vi "FlexMag - 23-03-2023.vi"() -> ()   [LabVIEW 2018] (continued)
            # "Cheksum 3 haneli olmalı"
            # "Address"
            n5110 = Concatenate Strings("003" ("write buffer"), "10" ("string"), "010" ("string"), "06" ("string"), "000000" ("string")) -> (w9122:string)
            n5111 = String To Byte Array(string=w9122) -> (unsigned byte array=w9127:u8[])
            n5112 = for {
              tunnel: w9127 -> [w9148] mode=indexing
              shift-right: [w9146] -> w9129
              shift-left: u8 0 -> [w9147]
              n5113 = Add(x=w9148, y=w9147) -> (x+y=w9146:u8)
            }
            n5114 = Number To Decimal String(number=w9129) -> (decimal integer string=w9124:string)  [unwired: 1 in]
            n5115 = local write "Tp3 auto stop"(FALSE ("Tp3_auto_stop")) -> ()
            n5116 = String Length(string=w9124) -> (length=w9125:i32)
            n5117 = case shown="0, Default" w9125 {
              tunnel: w9124 -> [_ w9141 w9144 w9145]
              tunnel: ["" w9139 w9142 w9145] -> w9123
              frame 0, Default {
              }
              frame 1 {
                n5118 = Concatenate Strings("00" ("string"), w9141) -> (w9139:string)
              }
              frame 2 {
                n5119 = Concatenate Strings("0" ("string"), w9144) -> (w9142:string)
              }
              frame 3 {
              }
            }
            n5120 = Concatenate Strings(w9122, w9123, "\r") -> (w9119:string)
            n5121 = VISA Write(VISA resource name=w9118, write buffer=w9119, error in (no error)=w9117) -> (VISA resource name out=w9121:refnum<visa-resource-name>, error out=w9120:errorcluster)  [unwired: 1 out]
            n5122 = stacked-sequence {
              tunnel: [w9137] -> w9114
              tunnel: w9121 -> [w9137]
              tunnel: [w9136] -> w9113
              tunnel: w9120 -> [w9136]
              frame #0 {
                n5123 = Wait (ms)(milliseconds to wait=u32 100) -> ()  [unwired: 1 out]
              }
            }
            "Tp3_stop_cmnd" <- TRUE ("Tp3_stop_cmnd")
          }
          frame 3 {
            # "Cheksum 3 haneli olmalı"
            # "Address"
            n5124 = Multiply(x="Low_speed_value 3", y=ext 10.0) -> (x*y=w9156:ext)
            n5125 = To Unsigned Long Integer(number=w9156) -> (unsigned 32bit integer=w9155:u32)
            n5126 = Number To Decimal String(number=w9155) -> (decimal integer string=w9153:string)  [unwired: 1 out]
            n5127 = String Length(string=w9153) -> (length=w9154:i32)
            n5128 = case shown="0, Default" w9154 {
              tunnel: w9153 -> [_ w9180 w9183 w9184]
              tunnel: ["" w9179 w9182 w9184] -> w9152
              frame 0, Default {
              }
              frame 1 {
                n5129 = Concatenate Strings(w9180, "00" ("string")) -> (w9179:string)
              }
              frame 2 {
                n5130 = Concatenate Strings(w9183, "0" ("string")) -> (w9182:string)
              }
              frame 3 {
              }
            }
            n5131 = Concatenate Strings("003" ("write buffer"), "10" ("string"), "707" ("string"), "06" ("string"), "00" ("string"), w9152) -> (w9164:string)
            n5132 = String To Byte Array(string=w9164) -> (unsigned byte array=w9169:u8[])
            n5133 = for {
              tunnel: w9169 -> [w9198] mode=indexing
              shift-right: [w9196] -> w9171
              shift-left: u8 0 -> [w9197]
              n5134 = Add(x=w9198, y=w9197) -> (x+y=w9196:u8)
            }
            n5135 = Number To Decimal String(number=w9171) -> (decimal integer string=w9166:string)  [unwired: 1 in]
            n5136 = String Length(string=w9166) -> (length=w9167:i32)
            n5137 = case shown="0, Default" w9167 {
              tunnel: w9166 -> [_ w9191 w9194 w9195]
              tunnel: ["" w9189 w9192 w9195] -> w9165
              frame 0, Default {
              }
              frame 1 {
                n5138 = Concatenate Strings("00" ("string"), w9191) -> (w9189:string)
              }
              frame 2 {
                n5139 = Concatenate Strings("0" ("string"), w9194) -> (w9192:string)
              }
              frame 3 {
              }
            }
            n5140 = Concatenate Strings(w9164, w9165, "\r") -> (w9161:string)
            n5141 = VISA Write(VISA resource name=w9160, write buffer=w9161, error in (no error)=w9159) -> (VISA resource name out=w9163:refnum<visa-resource-name>, error out=w9162:errorcluster)  [unwired: 1 out]
            n5142 = local write "Tp3 auto set speed"(FALSE ("Tp3_auto_set_speed")) -> ()
            n5143 = stacked-sequence {
              tunnel: [w9187] -> w9151
              tunnel: w9163 -> [w9187]
              tunnel: [w9186] -> w9150
              tunnel: w9162 -> [w9186]
              frame #0 {
                n5144 = Wait (ms)(milliseconds to wait=u32 100) -> ()  [unwired: 1 out]
              }
            }
          }
          frame 4 {
            # "Cheksum 3 haneli olmalı"
            # "Address"
            n5145 = Concatenate Strings("003" ("write buffer"), "10" ("string"), "026" ("string"), "03" ("string"), "001" ("string")) -> (w9207:string)
            n5146 = String To Byte Array(string=w9207) -> (unsigned byte array=w9212:u8[])
            n5147 = for {
              tunnel: w9212 -> [w9233] mode=indexing
              shift-right: [w9231] -> w9214
              shift-left: u8 0 -> [w9232]
              n5148 = Add(x=w9233, y=w9232) -> (x+y=w9231:u8)
            }
            n5149 = Number To Decimal String(number=w9214) -> (decimal integer string=w9209:string)  [unwired: 1 in]
            n5150 = String Length(string=w9209) -> (length=w9210:i32)
            n5151 = case shown="0, Default" w9210 {
              tunnel: w9209 -> [_ w9226 w9229 w9230]
              tunnel: ["" w9224 w9227 w9230] -> w9208
              frame 0, Default {
              }
              frame 1 {
                n5152 = Concatenate Strings("00" ("string"), w9226) -> (w9224:string)
              }
              frame 2 {
                n5153 = Concatenate Strings("0" ("string"), w9229) -> (w9227:string)
              }
              frame 3 {
              }
            }
            n5154 = local write "Tp3 auto low speed"(FALSE) -> ()
            n5155 = Concatenate Strings(w9207, w9208, "\r") -> (w9204:string)
            n5156 = VISA Write(VISA resource name=w9203, write buffer=w9204, error in (no error)=w9202) -> (VISA resource name out=w9206:refnum<visa-resource-name>, error out=w9205:errorcluster)  [unwired: 1 out]
            n5157 = stacked-sequence {
              tunnel: [w9222] -> w9201
              tunnel: w9206 -> [w9222]
              tunnel: [w9221] -> w9200
              tunnel: w9205 -> [w9221]
              frame #0 {
                n5158 = Wait (ms)(milliseconds to wait=u32 100) -> ()  [unwired: 1 out]
              }
            }
          }
          frame 5 {
            # "Cheksum 3 haneli olmalı"
            # "Address"
            n5159 = Concatenate Strings("003" ("write buffer"), "10" ("string"), "026" ("string"), "03" ("string"), "000" ("string")) -> (w9242:string)
            n5160 = String To Byte Array(string=w9242) -> (unsigned byte array=w9247:u8[])
            n5161 = for {
              tunnel: w9247 -> [w9268] mode=indexing
              shift-right: [w9266] -> w9249
              shift-left: u8 0 -> [w9267]
              n5162 = Add(x=w9268, y=w9267) -> (x+y=w9266:u8)
            }
            n5163 = local write "Tp3 auto normal speed"(FALSE ("Tp3_auto_normal_speed")) -> ()
            n5164 = Number To Decimal String(number=w9249) -> (decimal integer string=w9244:string)  [unwired: 1 in]
            n5165 = String Length(string=w9244) -> (length=w9245:i32)
            n5166 = case shown="0, Default" w9245 {
              tunnel: w9244 -> [_ w9261 w9264 w9265]
              tunnel: ["" w9259 w9262 w9265] -> w9243
              frame 0, Default {
              }
              frame 1 {
                n5167 = Concatenate Strings("00" ("string"), w9261) -> (w9259:string)
              }
              frame 2 {
                n5168 = Concatenate Strings("0" ("string"), w9264) -> (w9262:string)
              }
              frame 3 {
              }
            }
            n5169 = Concatenate Strings(w9242, w9243, "\r") -> (w9239:string)
            n5170 = VISA Write(VISA resource name=w9238, write buffer=w9239, error in (no error)=w9237) -> (VISA resource name out=w9241:refnum<visa-resource-name>, error out=w9240:errorcluster)  [unwired: 1 out]
            n5171 = stacked-sequence {
              tunnel: [w9257] -> w9236
              tunnel: w9241 -> [w9257]
              tunnel: [w9256] -> w9235
              tunnel: w9240 -> [w9256]
              frame #0 {
                n5172 = Wait (ms)(milliseconds to wait=u32 100) -> ()  [unwired: 1 out]
              }
            }
          }
          frame 6 {
            # "Cheksum 3 haneli olmalı"
            # "Address"
            n5173 = Concatenate Strings("003" ("write buffer"), "10" ("string"), "023" ("string"), "06" ("string"), "111111" ("string")) -> (w9276:string)
            n5174 = String To Byte Array(string=w9276) -> (unsigned byte array=w9281:u8[])
            n5175 = for {
              tunnel: w9281 -> [w9302] mode=indexing
              shift-right: [w9300] -> w9283
              shift-left: u8 0 -> [w9301]
              n5176 = Add(x=w9302, y=w9301) -> (x+y=w9300:u8)
            }
            n5177 = Number To Decimal String(number=w9283) -> (decimal integer string=w9278:string)  [unwired: 1 in]
            n5178 = String Length(string=w9278) -> (length=w9279:i32)
            n5179 = case shown="0, Default" w9279 {
              tunnel: w9278 -> [_ w9295 w9298 w9299]
              tunnel: ["" w9293 w9296 w9299] -> w9277
              frame 0, Default {
              }
              frame 1 {
                n5180 = Concatenate Strings("00" ("string"), w9295) -> (w9293:string)
              }
              frame 2 {
                n5181 = Concatenate Strings("0" ("string"), w9298) -> (w9296:string)
              }
              frame 3 {
              }
            }
            n5182 = Concatenate Strings(w9276, w9277, "\r") -> (w9273:string)
            n5183 = VISA Write(VISA resource name=w9272, write buffer=w9273, error in (no error)=w9271) -> (VISA resource name out=w9275:refnum<visa-resource-name>, error out=w9274:errorcluster)  [unwired: 1 out]
            n5184 = stacked-sequence {
              tunnel: [w9291] -> w9270
              tunnel: w9275 -> [w9291]
              tunnel: [w9290] -> w9269
              tunnel: w9274 -> [w9290]
              frame #0 {
                n5185 = Wait (ms)(milliseconds to wait=u32 100) -> ()  [unwired: 1 out]
              }
            }
          }
          frame 7 {
            # "Cheksum 3 haneli olmalı"
            # "Address"
            n5186 = Concatenate Strings("003" ("write buffer"), "10" ("string"), "023" ("string"), "06" ("string"), "000000" ("string")) -> (w9310:string)
            n5187 = String To Byte Array(string=w9310) -> (unsigned byte array=w9315:u8[])
            n5188 = for {
              tunnel: w9315 -> [w9336] mode=indexing
              shift-right: [w9334] -> w9317
              shift-left: u8 0 -> [w9335]
              n5189 = Add(x=w9336, y=w9335) -> (x+y=w9334:u8)
            }
            n5190 = Number To Decimal String(number=w9317) -> (decimal integer string=w9312:string)  [unwired: 1 in]
            n5191 = String Length(string=w9312) -> (length=w9313:i32)
            n5192 = case shown="0, Default" w9313 {
              tunnel: w9312 -> [_ w9329 w9332 w9333]
              tunnel: ["" w9327 w9330 w9333] -> w9311
              frame 0, Default {
              }
              frame 1 {
                n5193 = Concatenate Strings("00" ("string"), w9329) -> (w9327:string)
              }
              frame 2 {
                n5194 = Concatenate Strings("0" ("string"), w9332) -> (w9330:string)
              }
              frame 3 {
              }
            }
            n5195 = Concatenate Strings(w9310, w9311, "\r") -> (w9307:string)
            n5196 = VISA Write(VISA resource name=w9306, write buffer=w9307, error in (no error)=w9305) -> (VISA resource name out=w9309:refnum<visa-resource-name>, error out=w9308:errorcluster)  [unwired: 1 out]
            n5197 = stacked-sequence {
              tunnel: [w9325] -> w9304
              tunnel: w9309 -> [w9325]
              tunnel: [w9324] -> w9303
              tunnel: w9308 -> [w9324]
              frame #0 {
                n5198 = Wait (ms)(milliseconds to wait=u32 100) -> ()  [unwired: 1 out]
              }
            }
          }
        }
      }
      frame #3 {
        n5199 = Or(x="Tp4 low speed gui", y="Tp4 auto low speed") -> (x .or. y?=w9351:bool)
        n5200 = Or(x="Tp4 set speed gui", y="Tp4 auto set speed") -> (x .or. y?=w9354:bool)
        n5201 = Or(x="Tp4 normal speed gui", y="Tp4 auto normal speed") -> (x .or. y?=w9348:bool)
        n5202 = Compound Arithmetic op=OR("Tp4 stop gui", "Tp4 stop gui 1", "Tp4 auto stop") -> (w9339:bool)
        n5203 = Compound Arithmetic op=OR("Tp4 start gui", "Tp4 start gui 1", "Tp4 auto start") -> (w9338:bool)
        n5204 = case shown="True" w9338 {
          tunnel: [FALSE w9367] -> w9337
          frame False {
          }
          frame True {
            n5205 = case shown="False" "tp4 start safety" {
              tunnel: [FALSE TRUE] -> w9367
              frame False {
                n5206 = local write "Tp4 auto start"(FALSE ("Tp1_auto_start")) -> ()
                n5207 = local write "Warning Message"("CH4 TP cannot be started." ("Error Message")) -> ()
              }
              frame True {
              }
            }
          }
        }
        n5208 = Build Array(FALSE, w9337, w9339, w9354, w9351, w9348, "Tp4 start initial", "Tp4 stop initial") -> (w9358:bool[])
        n5209 = Boolean Array To Number(Boolean array=w9358) -> (number=w9364:u32)
        n5210 = Mantissa & Exponent(0:w9364) -> (2:w9363:dbl)  [unwired: 1 out]
        n5211 = case shown="0, Default" w9363 {
          tunnel: w9362 -> [w9372 w9487 w9523 w9565 w9608 w9643 w9677 w9711]
          tunnel: w9361 -> [w9373 w9486 w9522 w9564 w9607 w9642 w9676 w9710]
          tunnel: [w9375 w9485 w9521 w9563 w9606 w9641 w9675 w9709] -> w9360
          tunnel: [w9374 w9484 w9520 w9562 w9605 w9640 w9674 w9708] -> w9359
          frame 0, Default {
            n5212 = stacked-sequence {
              seq-local: [w9381 _] -> [_ w9439]
              seq-local: [w9380 _] -> [_ w9440]
              tunnel: w9372 -> [w9391 _]
              tunnel: w9373 -> [w9390 _]
              tunnel: [_ w9442] -> w9375
              tunnel: [_ w9441] -> w9374
              frame #0 {
                # "Address"
                # "Cheksum 3 haneli olmalı"
                # "Address"
                n5213 = Concatenate Strings("004" ("write buffer"), "00" ("string"), "309" ("string"), "02" ("string"), "=?" ("string")) -> (w9400:string)
                n5214 = String To Byte Array(string=w9400) -> (unsigned byte array=w9405:u8[])
                n5215 = for {
                  tunnel: w9405 -> [w9437] mode=indexing
                  shift-right: [w9435] -> w9407
                  shift-left: u8 0 -> [w9436]
                  n5216 = Add(x=w9437, y=w9436) -> (x+y=w9435:u8)
                }
                n5217 = Number To Decimal String(number=w9407) -> (decimal integer string=w9402:string)  [unwired: 1 in]
                n5218 = String Length(string=w9402) -> (length=w9403:i32)
                n5219 = case shown="0, Default" w9403 {
                  tunnel: w9402 -> [_ w9430 w9433 w9434]
                  tunnel: ["" w9428 w9431 w9434] -> w9401
                  frame 0, Default {
                  }
                  frame 1 {
                    n5220 = Concatenate Strings("00" ("string"), w9430) -> (w9428:string)
                  }
                  frame 2 {
                    n5221 = Concatenate Strings("0" ("string"), w9433) -> (w9431:string)
                  }
                  frame 3 {
                  }
                }
                n5222 = Concatenate Strings(w9400, w9401, "\r") -> (w9392:string)
                n5223 = VISA Write(VISA resource name=w9391, write buffer=w9392, error in (no error)=w9390) -> (VISA resource name out=w9395:refnum<visa-resource-name>, error out=w9394:errorcluster)  [unwired: 1 out]
                n5224 = stacked-sequence {
                  tunnel: [w9426] -> w9397
                  tunnel: w9395 -> [w9426]
                  tunnel: [w9425] -> w9396
                  tunnel: w9394 -> [w9425]
                  frame #0 {
                    n5225 = Wait (ms)(milliseconds to wait=u32 100) -> ()  [unwired: 1 out]
                  }
                }
                n5226 = property class="Instr"(reference=w9397, error in=w9396) -> (reference out=w9399:refnum<visa-resource-name>, error out=w9398:errorcluster, "Serial Settings:Number of Bytes at Serial Port"=w9393:u32)
                n5227 = VISA Read(VISA resource name=w9399, byte count=w9393, error in (no error)=w9398) -> (VISA resource name out=w9381:refnum<visa-resource-name>, read buffer=w9388:string, error out=w9380:errorcluster)  [unwired: 1 out]
                n5228 = String Length(string=w9388) -> (length=w9389:i32)
                n5229 = Not Equal To 0?(x=w9389) -> (x != 0?=w9376:bool)
                n5230 = Concatenate Strings("004" ("regular expression"), "1030906" ("regular expression")) -> (w9387:string)
                n5231 = feedback #145() -> (w9378:bool)  [unwired: 1 in]
                n5232 = Match Pattern(string=w9388, regular expression=w9387) -> (after substring=w9382:string)  [unwired: 4 out]
                n5233 = case shown="True" w9376 {
                  tunnel: [FALSE w9417] -> w9377
                  tunnel: [TRUE FALSE] -> w9379
                  tunnel: w9378 -> [_ w9415]
                  frame False {
                  }
                  frame True {
                    n5234 = call "Elapsed Time40"("Reset"=w9415) -> ("Elapsed Time (s)"=w9418:dbl)  [unwired: 11 in, 7 out]
                    n5235 = Greater?(x=w9418, y=5.0) -> (0:w9417:bool)
                  }
                }
                "tp4 com" <- w9377
                n5236 = feedback-in #145(w9379) -> ()
                n5237 = String Length(string=w9382) -> (length=w9384:i32)
                n5238 = Not Equal To 0?(x=w9384) -> (x != 0?=w9383:bool)
                n5239 = case shown="True" w9383 {
                  tunnel: w9382 -> [_ w9420]
                  frame False {
                  }
                  frame True {
                    n5240 = String Subset(string=w9420, length (rest)=6 ("length (rest)")) -> (substring=w9422:string)  [unwired: 1 out]
                    n5241 = Decimal String To Number(string=w9422) -> (number=→"Tp4 speed gui":i32)  [unwired: 3 out]
                    "tp4 readout" <- w9420
                  }
                }
              }
              frame #1 {
                # "Address"
                # "Cheksum 3 haneli olmalı"
                # "Address"
                n5242 = Concatenate Strings("004" ("write buffer"), "00" ("string"), "307" ("string"), "02" ("string"), "=?" ("string")) -> (w9455:string)
                n5243 = String To Byte Array(string=w9455) -> (unsigned byte array=w9460:u8[])
                n5244 = for {
                  tunnel: w9460 -> [w9481] mode=indexing
                  shift-right: [w9479] -> w9462
                  shift-left: u8 0 -> [w9480]
                  n5245 = Add(x=w9481, y=w9480) -> (x+y=w9479:u8)
                }
                n5246 = Number To Decimal String(number=w9462) -> (decimal integer string=w9457:string)  [unwired: 1 in]
                n5247 = String Length(string=w9457) -> (length=w9458:i32)
                n5248 = case shown="0, Default" w9458 {
                  tunnel: w9457 -> [_ w9474 w9477 w9478]
                  tunnel: ["" w9472 w9475 w9478] -> w9456
                  frame 0, Default {
                  }
                  frame 1 {
                    n5249 = Concatenate Strings("00" ("string"), w9474) -> (w9472:string)
                  }
                  frame 2 {
                    n5250 = Concatenate Strings("0" ("string"), w9477) -> (w9475:string)
                  }
                  frame 3 {
                  }
                }
                n5251 = Concatenate Strings(w9455, w9456, "\r") -> (w9447:string)
                n5252 = VISA Write(VISA resource name=w9439, write buffer=w9447, error in (no error)=w9440) -> (VISA resource name out=w9450:refnum<visa-resource-name>, error out=w9449:errorcluster)  [unwired: 1 out]
                n5253 = stacked-sequence {
                  tunnel: [w9470] -> w9452
                  tunnel: w9450 -> [w9470]
                  tunnel: [w9469] -> w9451
                  tunnel: w9449 -> [w9469]
                  frame #0 {
                    n5254 = Wait (ms)(milliseconds to wait=u32 100) -> ()  [unwired: 1 out]
                  }
                }
                n5255 = property class="Instr"(reference=w9452, error in=w9451) -> (reference out=w9454:refnum<visa-resource-name>, error out=w9453:errorcluster, "Serial Settings:Number of Bytes at Serial Port"=w9448:u32)
                n5256 = VISA Read(VISA resource name=w9454, byte count=w9448, error in (no error)=w9453) -> (VISA resource name out=w9442:refnum<visa-resource-name>, read buffer=w9446:string, error out=w9441:errorcluster)  [unwired: 1 out]
                n5257 = Concatenate Strings("004" ("regular expression"), "1030706" ("regular expression")) -> (w9445:string)
                n5258 = Match Pattern(string=w9446, regular expression=w9445) -> (after substring=→"after substring 4":string)  [unwired: 4 out]
              }
            }
          }
          frame 1 {
            # "Cheksum 3 haneli olmalı"
            # "Address"
            n5259 = Concatenate Strings("004" ("write buffer"), "10" ("string"), "010" ("string"), "06" ("string"), "111111" ("string")) -> (w9491:string)
            n5260 = String To Byte Array(string=w9491) -> (unsigned byte array=w9496:u8[])
            n5261 = for {
              tunnel: w9496 -> [w9517] mode=indexing
              shift-right: [w9515] -> w9498
              shift-left: u8 0 -> [w9516]
              n5262 = Add(x=w9517, y=w9516) -> (x+y=w9515:u8)
            }
            n5263 = local write "Tp4 auto start"(FALSE ("Tp4_auto_start")) -> ()
            n5264 = Number To Decimal String(number=w9498) -> (decimal integer string=w9493:string)  [unwired: 1 in]
            n5265 = String Length(string=w9493) -> (length=w9494:i32)
            n5266 = case shown="0, Default" w9494 {
              tunnel: w9493 -> [_ w9510 w9513 w9514]
              tunnel: ["" w9508 w9511 w9514] -> w9492
              frame 0, Default {
              }
              frame 1 {
                n5267 = Concatenate Strings("00" ("string"), w9510) -> (w9508:string)
              }
              frame 2 {
                n5268 = Concatenate Strings("0" ("string"), w9513) -> (w9511:string)
              }
              frame 3 {
              }
            }
            n5269 = local write "Tp4_stop_cmnd"(FALSE ("Tp4_stop_cmnd")) -> ()
            n5270 = Concatenate Strings(w9491, w9492, "\r") -> (w9488:string)
            n5271 = VISA Write(VISA resource name=w9487, write buffer=w9488, error in (no error)=w9486) -> (VISA resource name out=w9490:refnum<visa-resource-name>, error out=w9489:errorcluster)  [unwired: 1 out]
            n5272 = stacked-sequence {
              tunnel: [w9506] -> w9485
              tunnel: w9490 -> [w9506]
              tunnel: [w9505] -> w9484
              tunnel: w9489 -> [w9505]
              frame #0 {
                n5273 = Wait (ms)(milliseconds to wait=u32 100) -> ()  [unwired: 1 out]
              }
            }
          }
          frame 2 {
            # "Cheksum 3 haneli olmalı"
            # "Address"
            n5274 = Concatenate Strings("004" ("write buffer"), "10" ("string"), "010" ("string"), "06" ("string"), "000000" ("string")) -> (w9527:string)
            n5275 = String To Byte Array(string=w9527) -> (unsigned byte array=w9532:u8[])
            n5276 = for {
              tunnel: w9532 -> [w9553] mode=indexing
              shift-right: [w9551] -> w9534
              shift-left: u8 0 -> [w9552]
              n5277 = Add(x=w9553, y=w9552) -> (x+y=w9551:u8)
            }
            n5278 = local write "Tp4 auto stop"(FALSE ("Tp4_auto_stop")) -> ()
            n5279 = Number To Decimal String(number=w9534) -> (decimal integer string=w9529:string)  [unwired: 1 in]
            n5280 = String Length(string=w9529) -> (length=w9530:i32)
            n5281 = case shown="0, Default" w9530 {
              tunnel: w9529 -> [_ w9546 w9549 w9550]
              tunnel: ["" w9544 w9547 w9550] -> w9528
              frame 0, Default {
              }
              frame 1 {
                n5282 = Concatenate Strings("00" ("string"), w9546) -> (w9544:string)
              }
              frame 2 {
                n5283 = Concatenate Strings("0" ("string"), w9549) -> (w9547:string)
              }
              frame 3 {
              }
            }
            n5284 = Concatenate Strings(w9527, w9528, "\r") -> (w9524:string)
            n5285 = VISA Write(VISA resource name=w9523, write buffer=w9524, error in (no error)=w9522) -> (VISA resource name out=w9526:refnum<visa-resource-name>, error out=w9525:errorcluster)  [unwired: 1 out]
            n5286 = stacked-sequence {
              tunnel: [w9542] -> w9521
              tunnel: w9526 -> [w9542]
              tunnel: [w9541] -> w9520
              tunnel: w9525 -> [w9541]
              frame #0 {
                n5287 = Wait (ms)(milliseconds to wait=u32 100) -> ()  [unwired: 1 out]
              }
            }
            "Tp4_stop_cmnd" <- TRUE ("Tp4_stop_cmnd")
          }
          frame 3 {
            # "Address"
            n5288 = Multiply(x="Low_speed_value 4", y=ext 10.0) -> (x*y=w9559:ext)
            n5289 = To Unsigned Long Integer(number=w9559) -> (unsigned 32bit integer=w9558:u32)
            n5290 = Number To Decimal String(number=w9558) -> (decimal integer string=w9556:string)  [unwired: 1 out]
            n5291 = String Length(string=w9556) -> (length=w9557:i32)
            n5292 = case shown="0, Default" w9557 {
              tunnel: w9556 -> [_ w9585 w9588 w9589]
              tunnel: ["" w9584 w9587 w9589] -> w9555
              frame 0, Default {
              }
              frame 1 {
                n5293 = Concatenate Strings(w9585, "00" ("string")) -> (w9584:string)
              }
              frame 2 {
                n5294 = Concatenate Strings(w9588, "0" ("string")) -> (w9587:string)
              }
              frame 3 {
              }
            }
            n5295 = Concatenate Strings("004" ("write buffer"), "10" ("string"), "707" ("string"), "06" ("string"), "00" ("string"), w9555) -> (w9569:string)
            n5296 = String To Byte Array(string=w9569) -> (unsigned byte array=w9574:u8[])
            n5297 = for {
              tunnel: w9574 -> [w9603] mode=indexing
              shift-right: [w9601] -> w9576
              shift-left: u8 0 -> [w9602]
              n5298 = Add(x=w9603, y=w9602) -> (x+y=w9601:u8)
            }
            n5299 = Number To Decimal String(number=w9576) -> (decimal integer string=w9571:string)  [unwired: 1 in]
            n5300 = String Length(string=w9571) -> (length=w9572:i32)
            n5301 = case shown="0, Default" w9572 {
              tunnel: w9571 -> [_ w9596 w9599 w9600]
              tunnel: ["" w9594 w9597 w9600] -> w9570
              frame 0, Default {
              }
              frame 1 {
                n5302 = Concatenate Strings("00" ("string"), w9596) -> (w9594:string)
              }
              frame 2 {
                n5303 = Concatenate Strings("0" ("string"), w9599) -> (w9597:string)
              }
              frame 3 {
              }
            }
            n5304 = Concatenate Strings(w9569, w9570, "\r") -> (w9566:string)
            n5305 = VISA Write(VISA resource name=w9565, write buffer=w9566, error in (no error)=w9564) -> (VISA resource name out=w9568:refnum<visa-resource-name>, error out=w9567:errorcluster)  [unwired: 1 out]
            n5306 = stacked-sequence {
              tunnel: [w9592] -> w9563
              tunnel: w9568 -> [w9592]
              tunnel: [w9591] -> w9562
              tunnel: w9567 -> [w9591]
              frame #0 {
                n5307 = Wait (ms)(milliseconds to wait=u32 100) -> ()  [unwired: 1 out]
              }
            }
            n5308 = local write "Tp4 auto set speed"(FALSE ("Tp4_auto_set_speed")) -> ()
          }
          frame 4 {
            # "Cheksum 3 haneli olmalı"
            # "Address"
            n5309 = Concatenate Strings("004" ("write buffer"), "10" ("string"), "026" ("string"), "03" ("string"), "001" ("string")) -> (w9612:string)
            n5310 = String To Byte Array(string=w9612) -> (unsigned byte array=w9617:u8[])
            n5311 = for {
              tunnel: w9617 -> [w9638] mode=indexing
              shift-right: [w9636] -> w9619
              shift-left: u8 0 -> [w9637]
              n5312 = Add(x=w9638, y=w9637) -> (x+y=w9636:u8)
            }
            n5313 = local write "Tp4 auto low speed"(FALSE ("Tp4_auto_low_speed")) -> ()
            n5314 = Number To Decimal String(number=w9619) -> (decimal integer string=w9614:string)  [unwired: 1 in]
            n5315 = String Length(string=w9614) -> (length=w9615:i32)
            n5316 = case shown="0, Default" w9615 {
              tunnel: w9614 -> [_ w9631 w9634 w9635]
              tunnel: ["" w9629 w9632 w9635] -> w9613
              frame 0, Default {
              }
              frame 1 {
                n5317 = Concatenate Strings("00" ("string"), w9631) -> (w9629:string)
              }
              frame 2 {
                n5318 = Concatenate Strings("0" ("string"), w9634) -> (w9632:string)
              }
              frame 3 {
              }
            }
            n5319 = Concatenate Strings(w9612, w9613, "\r") -> (w9609:string)
            n5320 = VISA Write(VISA resource name=w9608, write buffer=w9609, error in (no error)=w9607) -> (VISA resource name out=w9611:refnum<visa-resource-name>, error out=w9610:errorcluster)  [unwired: 1 out]
            n5321 = stacked-sequence {
              tunnel: [w9627] -> w9606
              tunnel: w9611 -> [w9627]
              tunnel: [w9626] -> w9605
              tunnel: w9610 -> [w9626]
              frame #0 {
                n5322 = Wait (ms)(milliseconds to wait=u32 100) -> ()  [unwired: 1 out]
              }
            }
          }
          frame 5 {
            # "Cheksum 3 haneli olmalı"
            # "Address"
            n5323 = Concatenate Strings("004" ("write buffer"), "10" ("string"), "026" ("string"), "03" ("string"), "000" ("string")) -> (w9647:string)
            n5324 = String To Byte Array(string=w9647) -> (unsigned byte array=w9652:u8[])
            n5325 = for {
              tunnel: w9652 -> [w9673] mode=indexing
              shift-right: [w9671] -> w9654
              shift-left: u8 0 -> [w9672]
              n5326 = Add(x=w9673, y=w9672) -> (x+y=w9671:u8)
            }
            n5327 = Number To Decimal String(number=w9654) -> (decimal integer string=w9649:string)  [unwired: 1 in]
            n5328 = local write "Tp4 auto normal speed"(FALSE ("Tp4_auto_normal_speed")) -> ()
            n5329 = String Length(string=w9649) -> (length=w9650:i32)
            n5330 = case shown="0, Default" w9650 {
              tunnel: w9649 -> [_ w9666 w9669 w9670]
              tunnel: ["" w9664 w9667 w9670] -> w9648
              frame 0, Default {
              }
              frame 1 {
                n5331 = Concatenate Strings("00" ("string"), w9666) -> (w9664:string)
              }
              frame 2 {
                n5332 = Concatenate Strings("0" ("string"), w9669) -> (w9667:string)
              }
              frame 3 {
              }
            }
            n5333 = Concatenate Strings(w9647, w9648, "\r") -> (w9644:string)
            n5334 = VISA Write(VISA resource name=w9643, write buffer=w9644, error in (no error)=w9642) -> (VISA resource name out=w9646:refnum<visa-resource-name>, error out=w9645:errorcluster)  [unwired: 1 out]
            n5335 = stacked-sequence {
              tunnel: [w9662] -> w9641
              tunnel: w9646 -> [w9662]
              tunnel: [w9661] -> w9640
              tunnel: w9645 -> [w9661]
              frame #0 {
                n5336 = Wait (ms)(milliseconds to wait=u32 100) -> ()  [unwired: 1 out]
              }
            }
          }
          frame 6 {
            # "Cheksum 3 haneli olmalı"
            # "Address"
            n5337 = Concatenate Strings("004" ("write buffer"), "10" ("string"), "023" ("string"), "06" ("string"), "111111" ("string")) -> (w9681:string)
            n5338 = String To Byte Array(string=w9681) -> (unsigned byte array=w9686:u8[])
            n5339 = for {
              tunnel: w9686 -> [w9707] mode=indexing
              shift-right: [w9705] -> w9688
              shift-left: u8 0 -> [w9706]
              n5340 = Add(x=w9707, y=w9706) -> (x+y=w9705:u8)
            }
            n5341 = Number To Decimal String(number=w9688) -> (decimal integer string=w9683:string)  [unwired: 1 in]
            n5342 = String Length(string=w9683) -> (length=w9684:i32)
            n5343 = case shown="0, Default" w9684 {
              tunnel: w9683 -> [_ w9700 w9703 w9704]
              tunnel: ["" w9698 w9701 w9704] -> w9682
              frame 0, Default {
              }
              frame 1 {
                n5344 = Concatenate Strings("00" ("string"), w9700) -> (w9698:string)
              }
              frame 2 {
                n5345 = Concatenate Strings("0" ("string"), w9703) -> (w9701:string)
              }
              frame 3 {
              }
            }
            n5346 = Concatenate Strings(w9681, w9682, "\r") -> (w9678:string)
            n5347 = VISA Write(VISA resource name=w9677, write buffer=w9678, error in (no error)=w9676) -> (VISA resource name out=w9680:refnum<visa-resource-name>, error out=w9679:errorcluster)  [unwired: 1 out]
            n5348 = stacked-sequence {
              tunnel: [w9696] -> w9675
              tunnel: w9680 -> [w9696]
              tunnel: [w9695] -> w9674
              tunnel: w9679 -> [w9695]
              frame #0 {
                n5349 = Wait (ms)(milliseconds to wait=u32 100) -> ()  [unwired: 1 out]
              }
            }
          }
          frame 7 {
            # "Cheksum 3 haneli olmalı"
            # "Address"
            n5350 = Concatenate Strings("004" ("write buffer"), "10" ("string"), "023" ("string"), "06" ("string"), "000000" ("string")) -> (w9715:string)
            n5351 = String To Byte Array(string=w9715) -> (unsigned byte array=w9720:u8[])
            n5352 = for {
              tunnel: w9720 -> [w9741] mode=indexing
              shift-right: [w9739] -> w9722
              shift-left: u8 0 -> [w9740]
              n5353 = Add(x=w9741, y=w9740) -> (x+y=w9739:u8)
            }
            n5354 = Number To Decimal String(number=w9722) -> (decimal integer string=w9717:string)  [unwired: 1 in]
            n5355 = String Length(string=w9717) -> (length=w9718:i32)
            n5356 = case shown="0, Default" w9718 {
              tunnel: w9717 -> [_ w9734 w9737 w9738]
              tunnel: ["" w9732 w9735 w9738] -> w9716
              frame 0, Default {
              }
              frame 1 {
                n5357 = Concatenate Strings("00" ("string"), w9734) -> (w9732:string)
              }
              frame 2 {
                n5358 = Concatenate Strings("0" ("string"), w9737) -> (w9735:string)
              }
              frame 3 {
              }
            }
            n5359 = Concatenate Strings(w9715, w9716, "\r") -> (w9712:string)
            n5360 = VISA Write(VISA resource name=w9711, write buffer=w9712, error in (no error)=w9710) -> (VISA resource name out=w9714:refnum<visa-resource-name>, error out=w9713:errorcluster)  [unwired: 1 out]
            n5361 = stacked-sequence {
              tunnel: [w9730] -> w9709
              tunnel: w9714 -> [w9730]
              tunnel: [w9729] -> w9708
              tunnel: w9713 -> [w9729]
              frame #0 {
                n5362 = Wait (ms)(milliseconds to wait=u32 100) -> ()  [unwired: 1 out]
              }
            }
          }
        }
      }
    }
  }
  n5363 = while {
    tunnel: w70 -> [w9746]
    tunnel: w71 -> [w9745]
    tunnel: [w9744] -> w72
    tunnel: [w9743] -> w73
    i -> [w9742]
    stop <- FALSE stop-if-true
    n5364 = Wait Until Next ms Multiple(millisecond multiple=u32 300) -> ()  [unwired: 1 out]
    n5365 = stacked-sequence {
      tunnel: w9746 -> [w9801]
      tunnel: w9745 -> [w9779]
      tunnel: [w9778] -> w9744
      tunnel: [w9777] -> w9743
      tunnel: w9742 -> [w9785]
      frame #0 {
        n5366 = Compound Arithmetic op=OR("Dc_off", "Dc_auto_off", "Dc_off_2") -> (w9772:bool)
        n5367 = Compound Arithmetic op=OR("Dc_host_auto", "DC_host", "DC_host 2") -> (w9749:bool)
        n5368 = Compound Arithmetic op=OR("Dc_auto_set_zero", "Dc_set_zero", "Dc_set_zero 2") -> (w9769:bool)
        n5369 = Boolean To (0,1)(Boolean=w9772) -> (0, 1=w9781:i16)
        n5370 = Boolean To (0,1)(Boolean=w9749) -> (0, 1=w9780:i16)
        n5371 = Compound Arithmetic op=OR("Dc_auto_off_ramp_up", "DC_ramp_up", "DC_ramp_up 2") -> (w9770:bool)
        n5372 = Compound Arithmetic op=OR("Dc_auto_ramp_down", "DC_ramp_down", "DC_ramp_down 2") -> (w9771:bool)
        n5373 = Compound Arithmetic op=OR("Dc_on", "Dc_auto_on", "Dc_on_2") -> (w9773:bool)
        n5374 = Boolean To (0,1)(Boolean=w9769) -> (0, 1=w9805:i16)
        n5375 = Multiply(x=w9780, y=i16 1) -> (x*y=w9802:i16)
        n5376 = Boolean To (0,1)(Boolean="DC_auto_voltage_mode") -> (0, 1=w9789:i16)
        n5377 = Boolean To (0,1)(Boolean=w9770) -> (0, 1=w9799:i16)
        n5378 = Boolean To (0,1)(Boolean=w9771) -> (0, 1=w9796:i16)
        n5379 = Boolean To (0,1)(Boolean="DC_auto_power_mode") -> (0, 1=w9793:i16)
        n5380 = Multiply(x=w9781, y=i16 3) -> (x*y=w9810:i16)
        n5381 = Multiply(x=w9805, y=i16 5) -> (x*y=w9804:i16)
        n5382 = Multiply(x=w9789, y=i16 9) -> (x*y=w9788:i16)
        n5383 = Multiply(x=w9799, y=i16 6) -> (x*y=w9795:i16)
        n5384 = Multiply(x=w9796, y=i16 7) -> (x*y=w9794:i16)
        n5385 = Multiply(x=w9793, y=i16 8) -> (x*y=w9791:i16)
        n5386 = Compound Arithmetic op=OR("Dc_set_ch2", "Dc_set_ch3", "Dc_auto_set") -> (w9768:bool)
        n5387 = Boolean To (0,1)(Boolean=w9773) -> (0, 1=w9814:i16)
        n5388 = Boolean To (0,1)(Boolean=w9768) -> (0, 1=w9809:i16)
        n5389 = Multiply(x=w9814, y=i16 2) -> (x*y=w9812:i16)
        n5390 = Multiply(x=w9809, y=i16 4) -> (x*y=w9807:i16)
        n5391 = Compound Arithmetic op=ADD(w9802, w9812, w9810, w9807, w9804, w9795, w9794, w9791, w9788) -> (w9800:i16)
        n5392 = Quotient & Remainder(x=w9785, y=5) -> (x-y*floor(x/y)=w9783:i32)  [unwired: 1 out]
        n5393 = Equal To 0?(x=w9783) -> (x = 0?=w9782:bool)
        n5394 = case shown="3" w9800 {
          tunnel: w9801 -> [w9819 w9901 w9907 w9924 w9941 w9974 w10002 w10030 w10055 w10062]
          tunnel: w9779 -> [w9818 w9900 w9910 w9923 w9940 w9973 w10001 w10029 w10054 w10061]
          tunnel: [w9816 w9899 w9909 w9922 w9936 w9972 w10000 w10028 w10053 w10060] -> w9778
          tunnel: [w9815 w9898 w9908 w9921 w9935 w9971 w9999 w10027 w10052 w10059] -> w9777
          tunnel: w9782 -> [w9817 _ _ _ _ _ _ _ _ _]
          frame 0, Default {
            n5395 = case shown="False" w9817 {
              tunnel: w9819 -> [w9823 w9869]
              tunnel: w9818 -> [w9822 w9868]
              tunnel: [w9821 w9865] -> w9816
              tunnel: [w9820 w9866] -> w9815
              frame False {
                n5396 = VISA Write(VISA resource name=w9823, write buffer="\bキ", error in (no error)=w9822) -> (VISA resource name out=w9846:refnum<visa-resource-name>, error out=w9847:errorcluster)  [unwired: 1 out]
                n5397 = stacked-sequence {
                  tunnel: [w9863] -> w9844
                  tunnel: w9846 -> [w9863]
                  tunnel: [w9862] -> w9843
                  tunnel: w9847 -> [w9862]
                  frame #0 {
                    n5398 = Wait Until Next ms Multiple(millisecond multiple=u32 40) -> ()  [unwired: 1 out]
                  }
                }
                n5399 = property class="Instr"(reference=w9844, error in=w9843) -> (reference out=w9838:refnum<visa-resource-name>, error out=w9840:errorcluster, "Serial Settings:Number of Bytes at Serial Port"=w9839:u32)
                n5400 = VISA Read(VISA resource name=w9838, byte count=w9839, error in (no error)=w9840) -> (VISA resource name out=w9821:refnum<visa-resource-name>, read buffer=w9853:string, error out=w9820:errorcluster)  [unwired: 1 out]
                "read buffer" <- w9853
                n5401 = String Length(string=w9853) -> (length=w9852:i32)
                n5402 = Match Pattern(string=w9853, regular expression="¥") -> (after substring=w9825:string)  [unwired: 4 out]
                n5403 = Equal To 0?(x=w9852) -> (x = 0?=w9851:bool)
                n5404 = String Subset(string=w9825, length (rest)=2 ("length (rest)")) -> (substring=w9835:string)  [unwired: 1 out]
                n5405 = String To Byte Array(string=w9835) -> (unsigned byte array=w9841:u8[])
                n5406 = Index Array(array=w9841, index=1) -> (element=w9830:u8)
                n5407 = Index Array(array=w9841, index=0) -> (element=w9828:u8)
                n5408 = To Unsigned Long Integer(number=w9830) -> (unsigned 32bit integer=w9832:u32)
                n5409 = To Unsigned Long Integer(number=w9828) -> (unsigned 32bit integer=w9827:u32)
                n5410 = Multiply(x=256, y=w9832) -> (x*y=w9829:u32)
                n5411 = String Length(string=w9825) -> (length=w9842:i32)
                n5412 = Not Equal To 0?(x=w9842) -> (x != 0?=w9824:bool)
                n5413 = Add(x=w9829, y=w9827) -> (x+y=w9826:u32)
                n5414 = feedback #146() -> (w9849:bool)  [unwired: 1 in]
                n5415 = case shown="True" w9851 {
                  tunnel: [TRUE FALSE] -> w9850
                  tunnel: w9849 -> [_ w9860]
                  tunnel: [FALSE w9857] -> w9848
                  frame False {
                  }
                  frame True {
                    n5416 = call "Elapsed Time65"("Reset"=w9860) -> ("Elapsed Time (s)"=w9858:dbl)  [unwired: 11 in, 7 out]
                    n5417 = Greater?(x=w9858, y=6.0) -> (0:w9857:bool)
                  }
                }
                n5418 = feedback-in #146(w9850) -> ()
                n5419 = case shown="True" w9824 {
                  tunnel: w9826 -> [_ w9864]
                  frame False {
                  }
                  frame True {
                    "Actual DC Power" <- w9864
                    "Actual DC Power : 2" <- w9864
                  }
                }
                n5420 = local write "Dcps_fail"(w9848) -> ()
              }
              frame True {
                n5421 = VISA Write(VISA resource name=w9869, write buffer="\bΞ", error in (no error)=w9868) -> (VISA resource name out=w9892:refnum<visa-resource-name>, error out=w9893:errorcluster)  [unwired: 1 out]
                n5422 = stacked-sequence {
                  tunnel: [w9896] -> w9884
                  tunnel: w9892 -> [w9896]
                  tunnel: [w9895] -> w9885
                  tunnel: w9893 -> [w9895]
                  frame #0 {
                    n5423 = Wait Until Next ms Multiple(millisecond multiple=u32 40) -> ()  [unwired: 1 out]
                  }
                }
                n5424 = property class="Instr"(reference=w9884, error in=w9885) -> (reference out=w9871:refnum<visa-resource-name>, error out=w9872:errorcluster, "Serial Settings:Number of Bytes at Serial Port"=w9870:u32)
                n5425 = VISA Read(VISA resource name=w9871, byte count=w9870, error in (no error)=w9872) -> (VISA resource name out=w9865:refnum<visa-resource-name>, read buffer=w9891:string, error out=w9866:errorcluster)  [unwired: 1 out]
                n5426 = Match Pattern(string=w9891, regular expression="¦") -> (after substring=w9890:string)  [unwired: 4 out]
                n5427 = String Length(string=w9890) -> (length=w9886:i32)
                n5428 = String Subset(string=w9890, length (rest)=2 ("length (rest)")) -> (substring=w9875:string)  [unwired: 1 out]
                n5429 = Not Equal To 0?(x=w9886) -> (x != 0?=w9889:bool)
                n5430 = String To Byte Array(string=w9875) -> (unsigned byte array=w9887:u8[])
                n5431 = Index Array(array=w9887, index=1) -> (element=w9879:u8)
                n5432 = Index Array(array=w9887, index=0) -> (element=w9882:u8)
                n5433 = To Unsigned Long Integer(number=w9879) -> (unsigned 32bit integer=w9880:u32)
                n5434 = To Unsigned Long Integer(number=w9882) -> (unsigned 32bit integer=w9883:u32)
                n5435 = Multiply(x=256, y=w9880) -> (x*y=w9881:u32)
                n5436 = Add(x=w9881, y=w9883) -> (x+y=w9888:u32)
                n5437 = case shown="True" w9889 {
                  tunnel: w9888 -> [_ w9894]
                  frame False {
                  }
                  frame True {
                    # "Volt"
                    "Actual DC Volt :" <- w9894
                    "Actual DC Volt2" <- w9894
                  }
                }
              }
            }
          }
          frame 1 {
            # "Host kontrol"
            n5438 = flat-sequence {
              frame #0 {
                n5439 = Wait (ms)(milliseconds to wait=u32 100) -> ()  [unwired: 1 out]
              }
              frame #1 {
                n5440 = local write "Dc_host_auto"(FALSE ("Dc_host_auto")) -> ()
              }
            }
            n5441 = VISA Write(VISA resource name=w9901, write buffer="\t\u000e\u0002\u0005", error in (no error)=w9900) -> (VISA resource name out=w9899:refnum<visa-resource-name>, error out=w9898:errorcluster)  [unwired: 1 out]
          }
          frame 2 {
            n5442 = local read "Dcps_fail"() -> (w9905:bool)
            n5443 = case shown="True" "dcps on safety" {
              tunnel: ["\bキ" "\b\u0002\n"] -> w9911
              tunnel: w9905 -> [_ w9914]
              frame False {
                n5444 = local write "Warning Message"("DCPS cannot be on !\nCheck Safety Rules.. " ("Warning Message")) -> ()
              }
              frame True {
                n5445 = case shown="False" w9914 {
                  frame False {
                    "Dcps_is_on" <- TRUE ("Dcps_is_on")
                  }
                  frame True {
                  }
                }
              }
            }
            n5446 = flat-sequence {
              frame #0 {
                n5447 = Wait (ms)(milliseconds to wait=u32 100) -> ()  [unwired: 1 out]
              }
              frame #1 {
                n5448 = local write "Dc_auto_on"(FALSE ("Dc_auto_on")) -> ()
              }
            }
            n5449 = VISA Write(VISA resource name=w9907, write buffer=w9911, error in (no error)=w9910) -> (VISA resource name out=w9909:refnum<visa-resource-name>, error out=w9908:errorcluster)  [unwired: 1 out]
          }
          frame 3 {
            w9919 = 0.0 ("Dc_set_pow")
            n5450 = local write "Dc_auto_off"(FALSE ("Dc_auto_off")) -> ()
            n5451 = local write "Set DC Power ch2"(w9919) -> ()
            n5452 = local write "Set DC Power ch3"(w9919) -> ()
            n5453 = local write "Set DC Power auto"(w9919) -> ()
            n5454 = flat-sequence {
              frame #0 {
              }
              frame #1 {
                n5455 = local write "Dcps_is_on"(FALSE ("DC_auto_off")) -> ()
                n5456 = Wait (ms)(milliseconds to wait=u32 100) -> ()  [unwired: 1 out]
              }
            }
            n5457 = VISA Write(VISA resource name=w9924, write buffer="\b\u0001\t", error in (no error)=w9923) -> (VISA resource name out=w9922:refnum<visa-resource-name>, error out=w9921:errorcluster)  [unwired: 1 out]
          }
          frame 4 {
            w9937 = 2000.0 ("y")
            n5458 = local read "Dc_auto_set"() -> (w9929:bool)
            n5459 = local read "Dc_set_ch2"() -> (w9934:bool)
            n5460 = local read "Dc_set_ch3"() -> (w9933:bool)
            n5461 = case shown="True" w9933 {
              tunnel: [0.0 ("Set DC Power 2") "Set DC Power ch3"] -> w9930
              frame False {
              }
              frame True {
                n5462 = local write "Dc_set_ch3"(FALSE ("Dc_set")) -> ()
              }
            }
            n5463 = case shown="True" w9934 {
              tunnel: [0.0 ("Set DC Power") "Set DC Power ch2"] -> w9931
              frame False {
              }
              frame True {
                n5464 = local write "Dc_set_ch2"(FALSE ("Dc_set")) -> ()
              }
            }
            n5465 = case shown="True" w9929 {
              tunnel: [0.0 ("Set DC Power auto") "Set DC Power auto"] -> w9928
              frame False {
              }
              frame True {
                n5466 = local write "Dc_auto_set"(FALSE ("Dc_auto_set")) -> ()
              }
            }
            n5467 = flat-sequence {
              frame #0 {
                n5468 = Wait (ms)(milliseconds to wait=u32 300) -> ()  [unwired: 1 out]
              }
              frame #1 {
              }
            }
            n5469 = Compound Arithmetic op=ADD(w9928, w9931, w9930) -> (w9932:dbl)
            n5470 = Less Or Equal?(x=w9932, y=w9937) -> (x <= y?=w9938:bool)
            n5471 = Select(t=w9932, s=w9938, f=w9937) -> (s? t:f=w9939:dbl)
            n5472 = Quotient & Remainder(x=w9939, y=256.0) -> (x-y*floor(x/y)=w9956:dbl, floor(x/y)=w9955:dbl)
            n5473 = Build Array(w9956) -> (w9948:dbl[])
            n5474 = Build Array(w9955) -> (w9950:dbl[])
            n5475 = Byte Array To String(unsigned byte array=w9948) -> (string=w9949:string)
            n5476 = Byte Array To String(unsigned byte array=w9950) -> (string=w9951:string)
            n5477 = Concatenate Strings("\n\u0006", w9949, w9951) -> (w9946:string)
            n5478 = String To Byte Array(string=w9946) -> (unsigned byte array=w9942:u8[])
            n5479 = for {
              tunnel: w9942 -> [w9969] mode=indexing
              shift-right: [w9967] -> w9944
              shift-left: 0 -> [w9968]
              n5480 = Exclusive Or(1:w9968, 2:w9969) -> (0:w9967:i32)
            }
            n5481 = Build Array(w9944) -> (w9954:i32[])
            n5482 = Byte Array To String(unsigned byte array=w9954) -> (string=w9945:string)
            n5483 = Concatenate Strings(w9946, w9945) -> (w9952:string)
            n5484 = VISA Write(VISA resource name=w9941, write buffer=w9952, error in (no error)=w9940) -> (VISA resource name out=w9936:refnum<visa-resource-name>, error out=w9935:errorcluster)  [unwired: 1 out]
          }
          frame 5 {
            w9970 = 0.0 ("Dc_set_pow")
            n5485 = Quotient & Remainder(x=0.0, y=256.0) -> (x-y*floor(x/y)=w9989:dbl, floor(x/y)=w9988:dbl)
            n5486 = Build Array(w9989) -> (w9981:dbl[])
            n5487 = Build Array(w9988) -> (w9983:dbl[])
            n5488 = Byte Array To String(unsigned byte array=w9981) -> (string=w9982:string)
            n5489 = Byte Array To String(unsigned byte array=w9983) -> (string=w9984:string)
            n5490 = local write "Set DC Power ch2"(w9970) -> ()
            n5491 = local write "Set DC Power ch3"(w9970) -> ()
            n5492 = Concatenate Strings("\n\u0006", w9982, w9984) -> (w9979:string)
            n5493 = String To Byte Array(string=w9979) -> (unsigned byte array=w9975:u8[])
            n5494 = for {
              tunnel: w9975 -> [w9995] mode=indexing
              shift-right: [w9993] -> w9977
              shift-left: 0 -> [w9994]
              n5495 = Exclusive Or(1:w9994, 2:w9995) -> (0:w9993:i32)
            }
            n5496 = Build Array(w9977) -> (w9987:i32[])
            n5497 = Byte Array To String(unsigned byte array=w9987) -> (string=w9978:string)
            n5498 = Concatenate Strings(w9979, w9978) -> (w9985:string)
            n5499 = flat-sequence {
              frame #0 {
                n5500 = Wait (ms)(milliseconds to wait=u32 300) -> ()  [unwired: 1 out]
              }
              frame #1 {
                n5501 = local write "Dc_auto_set_zero"(FALSE ("Dc_auto_set_zero")) -> ()
              }
            }
            n5502 = VISA Write(VISA resource name=w9974, write buffer=w9985, error in (no error)=w9973) -> (VISA resource name out=w9972:refnum<visa-resource-name>, error out=w9971:errorcluster)  [unwired: 1 out]
          }
          frame 6 {
            n5503 = Or(x="DC_ramp_up_time :", y="DC_ramp_up_time : 2") -> (x .or. y?=w9996:i32)
            n5504 = Multiply(x=w9996, y=10.0) -> (x*y=w10006:dbl)
            n5505 = flat-sequence {
              frame #0 {
                n5506 = Wait (ms)(milliseconds to wait=u32 300) -> ()  [unwired: 1 out]
              }
              frame #1 {
                n5507 = local write "Dc_auto_off_ramp_up"(FALSE ("Dc_auto_off_ramp_up")) -> ()
              }
            }
            n5508 = To Unsigned Long Integer(number=w10006) -> (unsigned 32bit integer=w10003:u32)
            n5509 = Quotient & Remainder(x=w10003, y=u32 256) -> (x-y*floor(x/y)=w10009:u32, floor(x/y)=w10008:u32)
            n5510 = Build Array(w10009, w10008) -> (w10005:u32[])
            n5511 = Byte Array To String(unsigned byte array=w10005) -> (string=w10012:string)
            n5512 = Concatenate Strings("\n\u001f", w10012) -> (w10013:string)
            n5513 = String To Byte Array(string=w10013) -> (unsigned byte array=w10018:u8[])
            n5514 = for {
              tunnel: w10018 -> [w10023] mode=indexing
              shift-right: [w10021] -> w10016
              shift-left: 0 -> [w10022]
              n5515 = Exclusive Or(1:w10022, 2:w10023) -> (0:w10021:i32)
            }
            n5516 = Build Array(w10016) -> (w10004:i32[])
            n5517 = Byte Array To String(unsigned byte array=w10004) -> (string=w10014:string)
            n5518 = Concatenate Strings(w10013, w10014) -> (w10011:string)
            n5519 = VISA Write(VISA resource name=w10002, write buffer=w10011, error in (no error)=w10001) -> (VISA resource name out=w10000:refnum<visa-resource-name>, error out=w9999:errorcluster)  [unwired: 1 out]
          }
          frame 7 {
            n5520 = Or(x="DC_ramp_down_time: 2", y="DC_ramp_down_time:") -> (x .or. y?=w10024:i32)
            n5521 = Multiply(x=w10024, y=10.0) -> (x*y=w10034:dbl)
            n5522 = flat-sequence {
              frame #0 {
                n5523 = Wait (ms)(milliseconds to wait=u32 300) -> ()  [unwired: 1 out]
              }
              frame #1 {
                n5524 = local write "Dc_auto_ramp_down"(FALSE ("Dc_auto_ramp_down")) -> ()
              }
            }
            n5525 = To Unsigned Long Integer(number=w10034) -> (unsigned 32bit integer=w10031:u32)
            n5526 = Quotient & Remainder(x=w10031, y=u32 256) -> (x-y*floor(x/y)=w10037:u32, floor(x/y)=w10036:u32)
            n5527 = Build Array(w10037, w10036) -> (w10033:u32[])
            n5528 = Byte Array To String(unsigned byte array=w10033) -> (string=w10040:string)
            n5529 = Concatenate Strings("\n ", w10040) -> (w10041:string)
            n5530 = String To Byte Array(string=w10041) -> (unsigned byte array=w10046:u8[])
            n5531 = for {
              tunnel: w10046 -> [w10051] mode=indexing
              shift-right: [w10049] -> w10044
              shift-left: 0 -> [w10050]
              n5532 = Exclusive Or(1:w10050, 2:w10051) -> (0:w10049:i32)
            }
            n5533 = Build Array(w10044) -> (w10032:i32[])
            n5534 = Byte Array To String(unsigned byte array=w10032) -> (string=w10042:string)
            n5535 = Concatenate Strings(w10041, w10042) -> (w10039:string)
            n5536 = VISA Write(VISA resource name=w10030, write buffer=w10039, error in (no error)=w10029) -> (VISA resource name out=w10028:refnum<visa-resource-name>, error out=w10027:errorcluster)  [unwired: 1 out]
          }
          frame 8 {
            n5537 = flat-sequence {
              frame #0 {
                n5538 = Wait (ms)(milliseconds to wait=u32 100) -> ()  [unwired: 1 out]
              }
              frame #1 {
                n5539 = local write "DC_auto_power_mode"(FALSE ("DC_auto_power_mode")) -> ()
              }
            }
            n5540 = VISA Write(VISA resource name=w10055, write buffer="\t\u0003\u0006\f", error in (no error)=w10054) -> (VISA resource name out=w10053:refnum<visa-resource-name>, error out=w10052:errorcluster)  [unwired: 1 out]
          }
          frame 9 {